vi "Controle_Manip_Main_GUI_Backup2.vi"() -> ()   [LabVIEW 2019] (continued)
                  n486 = Index Array(array=w526, index=0) -> (element=w525:refnum<vi>)
                  n487 = property class="Page"(reference=w525, "PageVis"=w524) -> ()  [unwired: 1 in, 2 out]
                }
              }
            }
            frame #13 {
              # "Advance progress bar"
              n488 = local write "Scan Main Progess Bar"(u8 70 ("Scan Main Progess Bar")) -> ()
            }
            frame #14 {
              # "PZA12 Fine Delay Translation Stage"
              n489 = case shown="True" "PZC200 On?" {
                frame False {
                  n490 = local read "Scan Contrast Ctrls"() -> (w571:refnum<vi>[])
                  n491 = local read "ESP 301 On?"() -> (w570:bool)
                  n492 = call "Enable&Disable_Controls.vi"("Enum"=enum16{"Enabled", "Disabled", "Disabled&Grayed"}."Disabled&Grayed", "References"=w571) -> ()  [unwired: 1 in]
                  n493 = case shown="True" w570 {
                    frame True {
                      n494 = property on="Experimental parameters tab" class="TabCtl (strict)" props=["Pages", "Value"]() -> ("Pages"=w576:refnum<vi>[])  [unwired: 2 in, 3 out]
                      n495 = property on="Experiment Graph Controls" class="TabCtl (strict)" props=["Value", "Pages"]() -> ("Pages"=w577:refnum<vi>[])  [unwired: 2 in, 3 out]
                      n496 = Index Array(array=w576, index=3) -> (element=w575:refnum<vi>)
                      n497 = Index Array(array=w577, index=3) -> (element=w579:refnum<vi>)
                      n498 = property class="Page"(reference=w575, "PageVis"=TRUE ("Page Visible")) -> ()  [unwired: 1 in, 2 out]
                      n499 = property class="Page"(reference=w579, "PageVis"=TRUE ("Page Visible")) -> ()  [unwired: 1 in, 2 out]
                    }
                    frame False {
                      n500 = property on="Experimental parameters tab" class="TabCtl (strict)"() -> ("Pages"=w584:refnum<vi>[])  [unwired: 2 in, 2 out]
                      n501 = property on="Experiment Graph Controls" class="TabCtl (strict)" props=["Value", "Pages"]() -> ("Pages"=w585:refnum<vi>[])  [unwired: 2 in, 3 out]
                      n502 = Index Array(array=w584, index=3) -> (element=w583:refnum<vi>)
                      n503 = Index Array(array=w585, index=3) -> (element=w587:refnum<vi>)
                      n504 = property class="Page"(reference=w583, "PageVis"=FALSE ("Page Visible")) -> ()  [unwired: 1 in, 2 out]
                      n505 = property class="Page"(reference=w587, "PageVis"=FALSE ("Page Visible")) -> ()  [unwired: 1 in, 2 out]
                    }
                  }
                }
                frame True {
                  n506 = stacked-sequence {
                    frame #0 {
                      w604 = TRUE
                      w603 = FALSE
                      n507 = property on="Experiment Graph Controls" class="TabCtl (strict)"("Value"=T25."Contrast" ("Experiment Graph Controls")) -> ("Pages"=w599:refnum<vi>[])  [unwired: 2 in, 2 out]
                      n508 = property on="Experimental parameters tab" class="TabCtl (strict)"("Value"=T19."Translation" ("Experimental parameters tab")) -> ("Pages"=w598:refnum<vi>[])  [unwired: 2 in, 2 out]
                      n509 = local read "Log file"() -> (w594:string)
                      n510 = Index Array(array=w599, index=3) -> (element=w601:refnum<vi>)
                      n511 = Index Array(array=w598, index=3) -> (element=w595:refnum<vi>)
                      n512 = property class="Page"(reference=w601, "PageVis"=TRUE ("Page Visible")) -> ()  [unwired: 1 in, 2 out]
                      n513 = property on="Stop Contrast" class="Bool (strict)"("Visible"=w603) -> ()  [unwired: 2 in, 2 out]
                      n514 = property on="Pause Contrast" class="Bool (strict)"("Visible"=w603) -> ()  [unwired: 2 in, 2 out]
                      n515 = property class="Page"(reference=w595, "PageVis"=TRUE ("Page Visible")) -> ()  [unwired: 1 in, 2 out]
                      n516 = call "Write2LogFile.vi"("Add to log file"="Initialise communication with PZC", "Log file before"=w594, "Checkbox"=FALSE) -> ("Log file after"=w593:string)
                      n517 = local write "Log file"(w593) -> ()
                      n518 = local read "Scan Contrast Ctrls"() -> (w606:refnum<vi>[])
                      n519 = property on="Save Contrast" class="Bool (strict)"("Visible"=w604) -> ()  [unwired: 2 in, 2 out]
                      n520 = property on="Acquire Contrast" class="Bool (strict)"("Visible"=w604) -> ()  [unwired: 2 in, 2 out]
                      n521 = call "Enable&Disable_Controls.vi"("Enum"=enum16{"Enabled", "Disabled", "Disabled&Grayed"}."Enabled", "References"=w606) -> ()  [unwired: 1 in]
                    }
                    frame #1 {
                      # "RS232/10"
                      n522 = local read "PZC200 COM Port"() -> (w608:dbl)
                      n523 = call "Create Instrument Channel.vi"("XON/XOFF Handshaking(F)"=TRUE, "Baud Rate (38400)"=u32 19200, "COM Port (1)"=w608, "(T) - GPIB, F - RS232"=FALSE) -> ("Instrument Channel out"=w612:string)  [unwired: 5 in, 2 out]
                      n524 = call "SendCommand.vi"("Command"="1TS?", "Instrument Channel"=w612) -> ("Instrument Channel out"=w613:string)  [unwired: 8 in, 1 out]
                      n525 = call "ReadCommand.vi"("Disable MAV check (F)"=TRUE, "Instrument Channel"=w613) -> ("Response"=w614:string, "Instrument Channel out"=w607:string)  [unwired: 7 in, 1 out]
                      "Response" <- w614
                      n526 = String Length(string=w614) -> (length=w621:i32)
                      n527 = Subtract(x=w621, y=1) -> (x-y=w619:i32)
                      n528 = local write "PZC200 Instrument Channel"(w607) -> ()
                      n529 = String Subset(string=w614, offset (0)=w619) -> (substring=w618:string)  [unwired: 1 in]
                      n530 = case shown="\"@\", Default" w618 {
                        tunnel: [FALSE TRUE TRUE] -> w617
                        frame "@", Default {
                        }
                        frame "Q" {
                        }
                        frame "P" {
                        }
                      }
                      n531 = local write "LinTFine Motor On?"(w617) -> ()
                      n532 = call "PZCGetPos.vi"("Instrument Channel"=w607) -> ("Position"=w615:i32)  [unwired: 1 in, 2 out]
                      n533 = local write "PZC Position Readout (usteps)"(w615) -> ()
                    }
                  }
                }
              }
            }
            frame #15 {
              # "Advance progress bar"
              n534 = local write "Scan Main Progess Bar"(u8 85 ("Scan Main Progess Bar")) -> ()
            }
            frame #16 {
              # "Attocube ANC350 with 2 ANPx51 and 1 ANPz51"
              n535 = case shown="True" "Attocubes On?" {
                tunnel: [FALSE ("Page Visible") TRUE] -> w627
                frame False {
                }
                frame True {
                  n536 = stacked-sequence {
                    frame #0 {
                      n537 = control-ref of="Experimental parameters tab"() -> (w637:refnum<vi>)
                      n538 = property class="TabCtl (strict)"(reference=w637, "Value"=T19."Microscope objective") -> ()  [unwired: 1 in, 2 out]
                      n539 = local read "Log file"() -> (w641:string)
                      n540 = control-ref of="Tab Objective Sample"() -> (w639:refnum<vi>)
                      n541 = call "Write2LogFile.vi"("Add to log file"="Initialise communication with ANC350", "Log file before"=w641, "Checkbox"=FALSE) -> ("Log file after"=w642:string)
                      n542 = local write "Log file"(w642) -> ()
                      n543 = property class="TabCtl (strict)"(reference=w639, "Value"=T22."Sample piezo stack") -> ()  [unwired: 1 in, 2 out]
                      "ourDLL" <- path "C:/Users/manip/Documents/Controle_Manip_2020/subVIs/Attocubes/anc350v4.dll"
                    }
                    frame #1 {
                      w647 = u32 1 items=["None", "USB", "TCP", "All"] ("Interface types")
                      n544 = local read "ourDLL"() -> (w644:path)
                      n545 = call "ANC350v4_Discover.vi"("Path to *.DLL"=w644, "Interface types"=w647) -> ("ANC350v4 found"=w646:u32, "error ANC350v4_discover"=w645:errorcluster)  [unwired: 12 in]
                      n546 = case shown="1" w646 {
                        tunnel: w645 -> [_ w649]
                        tunnel: w644 -> [_ w648]
                        frame 0, Default {
                        }
                        frame 1 {
                          n547 = stacked-sequence {
                            seq-local: [w651 _] -> [_ w682]
                            seq-local: [w650 _] -> [_ w681]
                            tunnel: w649 -> [w668 _]
                            tunnel: w648 -> [w657 w680]
                            frame #0 {
                              w652 = u8 0 items=["1", "2", "3"] ("axis")
                              w655 = u8 2 items=["1", "2", "3"] ("axis")
                              w656 = u8 1 items=["1", "2", "3"] ("axis")
                              n548 = call "ANC350v4sub_Connect.vi"("Path to *.DLL"=w657, "deviceNumber"=0, "error in"=w668) -> ("ANC350v4_Handle_Out"=w664:u64, "error ANC350v4_Dis/Connect"=w667:errorcluster)  [unwired: 11 in]
                              n549 = call "ANC350v4_GetDeviceInfo.vi"("Path to *.DLL"=w657, "deviceNumber"=u32 0, "error in"=w667) -> ("connected"=→"ANC connected":bool, "Error_ANC350v4_getDeviceInfo"=w663:errorcluster)  [unwired: 5 in, 6 out]
                              n550 = call "ANC350v4_GetPosition.vi"("deviceHandle"=w664, "Path to *.DLL"=w657, "axis"=w652, "error in"=w663) -> ("deviceHandle"=w661:u64, "Position [µm | m°]"=w662:dbl, "error ANC350v4_getPosition"=w660:errorcluster)  [unwired: 8 in, 1 out]
                              n551 = local write "Att Pos Y"(w662) -> ()
                              n552 = call "ANC350v4_GetPosition.vi"("deviceHandle"=w661, "Path to *.DLL"=w657, "axis"=w656, "error in"=w660) -> ("deviceHandle"=w659:u64, "Position [µm | m°]"=w653:dbl, "error ANC350v4_getPosition"=w658:errorcluster)  [unwired: 8 in, 1 out]
                              n553 = local write "Att Pos X"(w653) -> ()
                              n554 = call "ANC350v4_GetPosition.vi"("deviceHandle"=w659, "Path to *.DLL"=w657, "axis"=w655, "error in"=w658) -> ("deviceHandle"=w651:u64, "Position [µm | m°]"=w654:dbl, "error ANC350v4_getPosition"=w650:errorcluster)  [unwired: 8 in, 1 out]
                              n555 = local write "Att Pos Z"(w654) -> ()
                            }
                            frame #1 {
                              w670 = u8 2 items=["1", "2", "3"] ("axis")
                              w671 = u8 1 items=["1", "2", "3"] ("axis")
                              w672 = u8 0 items=["1", "2", "3"] ("axis")
                              w679 = 0.1 ("TargetRange [µm | m°]")
                              # "Define Target resolution in um"
                              n556 = call "ANC350v4_SetTargetRange.vi"("deviceHandle"=w682, "Path to *.DLL"=w680, "axis"=w672, "TargetRange [µm | m°]"=w679, "error in"=w681) -> ("deviceHandle"=w678:u64, "error ANC350v4_setTargetRange"=w676:errorcluster)  [unwired: 8 in, 1 out]
                              n557 = call "ANC350v4_SetTargetRange.vi"("deviceHandle"=w678, "Path to *.DLL"=w680, "axis"=w671, "TargetRange [µm | m°]"=w679, "error in"=w676) -> ("deviceHandle"=w677:u64, "error ANC350v4_setTargetRange"=w675:errorcluster)  [unwired: 8 in, 1 out]
                              n558 = call "ANC350v4_SetTargetRange.vi"("deviceHandle"=w677, "Path to *.DLL"=w680, "axis"=w670, "TargetRange [µm | m°]"=w679, "error in"=w675) -> ("deviceHandle"=→"Att DeviceHandle":u64, "error ANC350v4_setTargetRange"=→"Att Error":errorcluster)  [unwired: 8 in, 1 out]
                            }
                          }
                        }
                      }
                    }
                  }
                }
              }
              n559 = control-ref of="Tab Objective Sample"() -> (w629:refnum<vi>)
              n560 = property class="TabCtl (strict)"(reference=w629) -> ("Pages"=w630:refnum<vi>[])  [unwired: 1 in, 2 out]
              n561 = Index Array(array=w630, index=1) -> (element=w631:refnum<vi>)
              n562 = property class="Page"(reference=w631, "PageVis"=w627) -> ()  [unwired: 1 in, 2 out]
            }
            frame #17 {
              # "Montana Cryostation s50"
              n563 = case shown="True" "Cryostation On?" {
                frame False {
                }
                frame True {
                  w698 = 10.0 ("y")
                  n564 = call "CryoConnect.vi"() -> ("connection ID"=w688:refnum<k5>)
                  "Cryostation ID" <- w688
                  n565 = local read "Log file"() -> (w687:string)
                  n566 = call "Write2LogFile.vi"("Add to log file"="Initialise communication with Cryostation", "Log file before"=w687, "Checkbox"=FALSE) -> ("Log file after"=w686:string)
                  n567 = local write "Log file"(w686) -> ()
                  n568 = call "GetCryoInfo.vi"("connection ID"=w688) -> ("User Stability"=w693:dbl, "User Temp"=w692:dbl, "connection ID out"=w694:refnum<k5>, "Sample Stability"=w691:dbl, "Sample Temp"=w695:dbl, "Platform Stability"=w690:dbl, "Platform Temp"=w689:dbl)  [unwired: 4 in]
                  n569 = local write "Cryo Platform Temp"(w689) -> ()
                  n570 = Multiply(x=w695, y=w698) -> (x*y=w696:dbl)
                  n571 = local write "Cryo Sample Stability"(w691) -> ()
                  n572 = local write "Cryostation ID"(w694) -> ()
                  n573 = local write "Cryo User Stability"(w693) -> ()
                  n574 = local write "Cryo Sample Temp"(w695) -> ()
                  n575 = local write "Cryo Platform Stability"(w690) -> ()
                  n576 = local write "Cryo User Temp"(w692) -> ()
                  n577 = Round To Nearest(number=w696) -> (nearest integer value=w697:dbl)
                  n578 = Divide(x=w697, y=w698) -> (x/y=w699:dbl)
                  n579 = local write "Temperature (K)"(w699) -> ()
                }
              }
            }
            frame #18 {
              # "PicoHarp"
              n580 = case shown="True" "PicoHarp On?" {
                frame False {
                  n581 = local write "Connected"(FALSE) -> ()
                }
                frame True {
                  n582 = local read "Log file"() -> (w711:string)
                  n583 = property on="Experiment Graph Controls" class="TabCtl (strict)"("Value"=T25."APDs" ("Experiment Graph Controls")) -> ("Pages"=w706:refnum<vi>[])  [unwired: 2 in, 2 out]
                  n584 = call "Write2LogFile.vi"("Add to log file"="Initialise communication with PicoHarp", "Log file before"=w711, "Checkbox"=FALSE) -> ("Log file after"=w710:string)
                  n585 = call "PH_Init.vi"() -> ("PH_Init_Data"=→"PH_Init_Data":T11)
                  n586 = local write "Log file"(w710) -> ()
                  n587 = Index Array(array=w706, index=4) -> (element=w707:refnum<vi>)
                  n588 = property class="Page"(reference=w707, "PageVis"=TRUE ("Page Visible")) -> ()  [unwired: 1 in, 2 out]
                  n589 = local write "Connected"(TRUE) -> ()
                }
              }
            }
            frame #19 {
              # "Final activation message"
              n590 = local read "Log file"() -> (w717:string)
              n591 = property on="Experiment Graph Controls" class="TabCtl (strict)"("Value"=T25."Settings" ("Experiment Graph Controls")) -> ()  [unwired: 2 in, 2 out]
              n592 = call "Write2LogFile.vi"("Add to log file"="All devices activated !", "Log file before"=w717, "Checkbox"=FALSE) -> ("Log file after"=w718:string)
              n593 = local write "Log file"(w718) -> ()
              n594 = local write "Scan Main Progess Bar"(u8 100 ("Scan Main Progess Bar")) -> ()
            }
            frame #20 {
              # "Autosave Init"
              n595 = local read "Auto< ?"() -> (w719:bool)
              n596 = case shown="True" w719 {
                frame False {
                  w720 = TRUE ("Visible")
                  n597 = property on="Save Spectrum N" class="Bool (strict)"("Visible"=w720) -> ()  [unwired: 2 in, 2 out]
                  n598 = property on="Save XY Map" class="Bool (strict)"("Visible"=w720) -> ()  [unwired: 2 in, 2 out]
                  n599 = property on="Save Spectrum" class="Bool (strict)"("Visible"=w720) -> ()  [unwired: 2 in, 2 out]
                  n600 = property on="Save PLE" class="Bool (strict)"("Visible"=w720) -> ()  [unwired: 2 in, 2 out]
                  n601 = property on="Save fPow" class="Bool (strict)"("Visible"=w720) -> ()  [unwired: 2 in, 2 out]
                  n602 = property on="Save Custom Diode Spectrum" class="Bool (strict)"("Visible"=w720) -> ()  [unwired: 2 in, 2 out]
                  n603 = property on="Save Michelson" class="Bool (strict)"("Visible"=w720) -> ()  [unwired: 2 in, 2 out]
                  n604 = property on="Save Polarisation" class="Bool (strict)"("Visible"=w720) -> ()  [unwired: 2 in, 2 out]
                  n605 = property on="Save Contrast" class="Bool (strict)"("Visible"=w720) -> ()  [unwired: 2 in, 2 out]
                }
                frame True {
                  w721 = FALSE ("Visible")
                  n606 = property on="Save Spectrum N" class="Bool (strict)"("Visible"=w721) -> ()  [unwired: 2 in, 2 out]
                  n607 = property on="Save XY Map" class="Bool (strict)"("Visible"=w721) -> ()  [unwired: 2 in, 2 out]
                  n608 = property on="Save Spectrum" class="Bool (strict)"("Visible"=w721) -> ()  [unwired: 2 in, 2 out]
                  n609 = property on="Save PLE" class="Bool (strict)"("Visible"=w721) -> ()  [unwired: 2 in, 2 out]
                  n610 = property on="Save fPow" class="Bool (strict)"("Visible"=w721) -> ()  [unwired: 2 in, 2 out]
                  n611 = property on="Save Polarisation" class="Bool (strict)"("Visible"=w721) -> ()  [unwired: 2 in, 2 out]
                  n612 = property on="Save Michelson" class="Bool (strict)"("Visible"=w721) -> ()  [unwired: 2 in, 2 out]
                  n613 = property on="Save Contrast" class="Bool (strict)"("Visible"=w721) -> ()  [unwired: 2 in, 2 out]
                  n614 = property on="Save Custom Diode Spectrum" class="Bool (strict)"("Visible"=w721) -> ()  [unwired: 2 in, 2 out]
                }
              }
            }
          }
        }
      }
    }
    frame #2 {
      # "Main Program"
      n615 = while {
        stop <- w873 stop-if-true
        # "Main loop with unique event structure handling nearly all events"
        n616 = event shown="[50] \"Fit?\": Mouse Down" {
          selector: _ -> [_ _ _ _ _ _ _ _ _ _ _ _ _ _ _ _ _ _ _ _ _ _ _ _ _ _ _ _ _ _ _ _ _ _ _ _ _ _ _ _ _ _ _ _ _ _ _ _ _ _ _ _ _ _]
          dyn-events: _ -> [_ _ _ _ _ _ _ _ _ _ _ _ _ _ _ _ _ _ _ _ _ _ _ _ _ _ _ _ _ _ _ _ _ _ _ _ _ _ _ _ _ _ _ _ _ _ _ _ _ _ _ _ _ _]
          timeout: 500 -> [_ _ _ _ _ _ _ _ _ _ _ _ _ _ _ _ _ _ _ _ _ _ _ _ _ _ _ _ _ _ _ _ _ _ _ _ _ _ _ _ _ _ _ _ _ _ _ _ _ _ _ _ _ _]
          tunnel: [_ _ _ _ _ _ _ _ _ _ _ _ _ _ _ _ _ _ _ _ _ _ _ _ _ _ _ _ _ _ _ _ _ _ _ _ _ _ _ _ _ _ _ _ _ _ _ _ w4486 _ _ _ _ _] -> w873
          event "Acquire Time Trace", "Acquire Polarisation", "Acquire XY Map", "Acquire Contrast", "Acquire Michelson", "Acquire Spectrum", "Fast Acq", "Acquire Custom Diode Spectrum", "Acquire fPow", "Acquire PLE": Mouse Down {
            # "FAILLE\naucune protection \nde teigger si ESP et \nPicoHarp mais pas LF"
            # "Launch an acquisition or an experiment"
            n617 = event-data() -> ("CtlRef"=w879:refnum<vi>)  [unwired: 1 in, 7 out]
            n618 = local read "LightField On?"() -> (w876:bool)
            n619 = local read "PicoHarp On?"() -> (w877:bool)
            n620 = local read "ESP 300 On?"() -> (w878:bool)
            n621 = And(x=w878, y=w877) -> (x .and. y?=w875:bool)
            n622 = Or(x=w876, y=w875) -> (x .or. y?=w874:bool)
            n623 = stacked-sequence {
              tunnel: w879 -> [w881 w2777]
              tunnel: w874 -> [w880 _]
              frame #0 {
                # "Actual measurements"
                n624 = case shown="True" w880 {
                  tunnel: w881 -> [_ w886]
                  frame False {
                    n625 = local read "Log file"() -> (w885:string)
                    n626 = call "Write2LogFile.vi"("Add to log file"="LightField not activated; cannot acquire", "Log file before"=w885, "Checkbox"=FALSE) -> ("Log file after"=w884:string)
                    n627 = local write "Log file"(w884) -> ()
                  }
                  frame True {
                    n628 = property class="Bool"(reference=w886) -> ("Label.Text"=w887:string)  [unwired: 1 in, 2 out]
                    n629 = case shown="\"Acquire PLE\"" w887 {
                      frame "Acquire Spectrum", Default {
                        n630 = stacked-sequence {
                          frame #0 {
                            # "background"
                            n631 = local read "Background taken?"() -> (w888:bool)
                            n632 = case shown="False" w888 {
                              frame False {
                                n633 = stacked-sequence {
                                tunnel: [_ _ w934] -> w889
                                frame #0 {
                                n634 = property on="CCD 1D Spectrum Main" class="XYGraph (strict)"("YScale.Offset"=0.0 ("Y Scale.Offset and Multiplier:Offset")) -> ()  [unwired: 2 in, 2 out]
                                }
                                frame #1 {
                                # "make sure shutter is closed"
                                n635 = local read "KCube Shutter On?"() -> (w920:bool)
                                n636 = control-ref of="Shutter Ctrls"() -> (w924:refnum<vi>)
                                n637 = property class="Ring (strict)"(reference=w924) -> ("Value"=w923:u16)  [unwired: 1 in, 2 out]
                                n638 = control-ref of="KCube Shutter Device Reference"() -> (w925:refnum<vi>)
                                n639 = Equal?(x=w923, y=u16 0) -> (x = y?=w921:bool)
                                n640 = case shown="False" w921 {
                                tunnel: w925 -> [w928 _]
                                tunnel: w924 -> [w927 _]
                                tunnel: w920 -> [w926 _]
                                frame False {
                                n641 = call "Shutter.vi"("KCube Shutter Device Reference 2"=w928, "Shutter Ctrls 2"=w927, "Shutter on?"=w926) -> ()
                                }
                                frame True {
                                }
                                }
                                }
                                frame #2 {
                                # "acquire"
                                n642 = local read "LightField Automation error out"() -> (w932:errorcluster)
                                n643 = local read "LightField Automation out"() -> (w933:refnum<class "LightField Automation.lvclass">)
                                n644 = local read "Accumulations"() -> (w929:dbl)
                                n645 = call "LFA_Capture.vi"("error in (no error)"=w932, "Frames"=w929, "LightField Automation in"=w933) -> ("error out"=w931:errorcluster, "Data"=w934:T26, "LightField Automation out"=w930:refnum<class "LightField Automation.lvclass">)  [unwired: 6 in]
                                n646 = local write "LightField Automation error out"(w931) -> ()
                                n647 = local write "LightField Automation out"(w930) -> ()
                                }
                                }
                                n648 = local read "Acq Mode"() -> (w890:T3)
                                n649 = case shown="\"Spectrum\", Default" w890 {
                                selector: w890 -> [w891 w909]
                                tunnel: w889 -> [w892 w910]
                                frame "Spectrum", Default {
                                n650 = stacked-sequence {
                                tunnel: w892 -> [_ w903 _ _]
                                tunnel: w891 -> [_ w901 _ _]
                                frame #0 {
                                n651 = property on="CCD 2D Image Main" class="IntGraph (strict)"("Visible"=FALSE) -> ()  [unwired: 2 in, 2 out]
                                n652 = property on="CCD 1D Spectrum Main" class="XYGraph (strict)"("Visible"=TRUE) -> ()  [unwired: 2 in, 2 out]
                                }
                                frame #1 {
                                n653 = local read "Wavelength calibration"() -> (w900:dbl[])
                                n654 = local read "CCD ROI"() -> (w896:T20)
                                n655 = Divide(x=1239.842, y=w900) -> (x/y=w898:dbl[])
                                n656 = call "PrepareData4Graph.vi"("Wavelength nm"=w898, "DataLF"=w903, "CCD ROI"=w896, "AcqMode"=w901, "Data type"=T30."Spectre") -> ("Spectrum"=w902:cluster{"Array 2":dbl[], "Array":dbl[]}, "PLInt out"=w895:dbl[])  [unwired: 2 in, 2 out]
                                n657 = local write "CCD 1D Spectrum Main"(w902) -> ()
                                n658 = local write "BackgroundSpec"(w895) -> ()
                                }
                                frame #2 {
                                n659 = local read "BackgroundSpec"() -> (w904:dbl[])
                                n660 = call-poly <vilib>:"Mean.vi"("X"=w904) -> ("mean"=w906:dbl)  [unwired: 1 out]
                                n661 = Negate(x=w906) -> (-x=w905:dbl)
                                n662 = property on="CCD 1D Spectrum Main" class="XYGraph (strict)"("YScale.Offset"=w905) -> ()  [unwired: 2 in, 2 out]
                                }
                                frame #3 {
                                n663 = local write "Background taken?"(TRUE ("Background taken?")) -> ()
                                n664 = property on="Background substract" class="Enum (strict)"("Value"=enum16{"None", "Shutter"}."None" ("Background substract")) -> ()  [unwired: 2 in, 2 out]
                                }
                                }
                                }
                                frame "Image" {
                                n665 = stacked-sequence {
                                tunnel: w910 -> [_ w918]
                                tunnel: w909 -> [_ w916]
                                frame #0 {
                                n666 = property on="CCD 1D Spectrum Main" class="XYGraph (strict)"("Visible"=FALSE) -> ()  [unwired: 2 in, 2 out]
                                n667 = property on="CCD 2D Image Main" class="IntGraph (strict)"("Visible"=TRUE) -> ()  [unwired: 2 in, 2 out]
                                }
                                frame #1 {
                                n668 = local read "Wavelength calibration"() -> (w917:dbl[])
                                n669 = local read "CCD ROI"() -> (w913:T20)
                                n670 = call "PrepareData4Graph.vi"("Wavelength nm"=w917, "DataLF"=w918, "CCD ROI"=w913, "AcqMode"=w916, "Data type"=T30."Spectre") -> ("Intensity Graph"=w915:dbl[][])  [unwired: 2 in, 3 out]
                                n671 = local write "CCD 2D Image Main"(w915) -> ()
                                }
                                }
                                }
                                }
                              }
                              frame True {
                              }
                            }
                          }
                          frame #1 {
                            # "measurement"
                            n672 = stacked-sequence {
                              frame #0 {
                                # "open shutter if closed"
                                n673 = control-ref of="KCube Shutter Device Reference"() -> (w937:refnum<vi>)
                                n674 = control-ref of="Shutter Ctrls"() -> (w936:refnum<vi>)
                                n675 = property class="Ring (strict)"(reference=w936) -> ("Value"=w938:u16)  [unwired: 1 in, 2 out]
                                n676 = local read "KCube Shutter On?"() -> (w941:bool)
                                n677 = Equal?(x=w938, y=u16 0) -> (x = y?=w940:bool)
                                n678 = property on="Experiment Graph Controls" class="TabCtl (strict)"("Value"=T25."Spectrum" ("Experiment Graph Controls")) -> ()  [unwired: 2 in, 2 out]
                                n679 = case shown="True" w940 {
                                tunnel: w937 -> [_ w944]
                                tunnel: w936 -> [_ w943]
                                tunnel: w941 -> [_ w942]
                                frame False {
                                }
                                frame True {
                                n680 = call "Shutter.vi"("KCube Shutter Device Reference 2"=w944, "Shutter Ctrls 2"=w943, "Shutter on?"=w942) -> ()
                                }
                                }
                              }
                              frame #1 {
                                # "set CCD ROI and acquire"
                                n681 = local read "LightField Automation error out"() -> (w953:errorcluster)
                                n682 = local read "LightField Automation out"() -> (w945:refnum<class "LightField Automation.lvclass">)
                                n683 = local read "CCD ROI"() -> (w952:T20)
                                n684 = local read "Accumulations"() -> (w949:dbl)
                                n685 = call "Adv_SetROI.vi"("error in (no error)"=w953, "ROI"=w952, "LightField Automation in"=w945) -> ("error out"=w950:errorcluster, "LightField Automation out"=w951:refnum<class "LightField Automation.lvclass">)  [unwired: 7 in]
                                n686 = call "LFA_Capture.vi"("error in (no error)"=w950, "Frames"=w949, "LightField Automation in"=w951) -> ("error out"=w948:errorcluster, "Data"=w947:T26, "LightField Automation out"=w946:refnum<class "LightField Automation.lvclass">)  [unwired: 6 in]
                                n687 = local write "LightField Automation out"(w946) -> ()
                                n688 = local write "LightField Automation error out"(w948) -> ()
                                n689 = local write "Data"(w947) -> ()
                              }
                              frame #2 {
                                # "close shutter"
                                n690 = local read "KCube Shutter On?"() -> (w956:bool)
                                n691 = control-ref of="KCube Shutter Device Reference"() -> (w955:refnum<vi>)
                                n692 = control-ref of="Shutter Ctrls"() -> (w954:refnum<vi>)
                                n693 = call "Shutter.vi"("KCube Shutter Device Reference 2"=w955, "Shutter Ctrls 2"=w954, "Shutter on?"=w956) -> ()
                              }
                              frame #3 {
                                # "Show data accordingly"
                                n694 = local read "Data"() -> (w957:T26)
                                n695 = local read "Acq Mode"() -> (w958:T3)
                                n696 = case shown="\"Spectrum\", Default" w958 {
                                selector: w958 -> [w959 w978]
                                tunnel: w957 -> [w960 w979]
                                frame "Spectrum", Default {
                                n697 = stacked-sequence {
                                tunnel: w960 -> [_ w976 _]
                                tunnel: w959 -> [_ w975 _]
                                frame #0 {
                                n698 = property on="CCD 1D Spectrum Main" class="XYGraph (strict)"("Visible"=TRUE) -> ()  [unwired: 2 in, 2 out]
                                n699 = property on="CCD 2D Image Main" class="IntGraph (strict)"("Visible"=FALSE) -> ()  [unwired: 2 in, 2 out]
                                }
                                frame #1 {
                                n700 = local read "Wavelength calibration"() -> (w974:dbl[])
                                n701 = local read "CCD ROI"() -> (w970:T20)
                                n702 = local read "BackgroundSpec"() -> (w964:dbl[])
                                n703 = Divide(x=1239.842, y=w974) -> (x/y=w972:dbl[])
                                n704 = call "PrepareData4Graph.vi"("BackgroundSpec"=w964, "Wavelength nm"=w972, "DataLF"=w976, "CCD ROI"=w970, "AcqMode"=w975, "Data type"=T30."Spectre") -> ("Spectrum"=w963:cluster{"Array 2":dbl[], "Array":dbl[]}, "PLInt out"=w968:dbl[])  [unwired: 1 in, 2 out]
                                n705 = control-ref of="Cnts"() -> (w969:refnum<vi>)
                                n706 = local read "Excitation Power (uW)"() -> (w966:dbl)
                                n707 = local write "CCD 1D Spectrum Main"(w963) -> ()
                                n708 = local read "Acq Time (ms)"() -> (w967:dbl)
                                n709 = local read "Display Mode"() -> (w965:u16)
                                n710 = call "2Cnts.vi"("Array Background"=w964, "Pow W"=w966, "AcqTime ms"=w967, "Cnts Ref"=w969, "Display Mode"=w965, "Array"=w968) -> ()  [unwired: 1 out]
                                }
                                frame #2 {
                                n711 = property on="Full scale" class="Bool (strict)"("Val(Sgnl)"=TRUE ("Value (Signaling)")) -> ()  [unwired: 2 in, 2 out]
                                }
                                }
                                }
                                frame "Image" {
                                n712 = stacked-sequence {
                                tunnel: w979 -> [_ w987]
                                tunnel: w978 -> [_ w985]
                                frame #0 {
                                n713 = property on="CCD 1D Spectrum Main" class="XYGraph (strict)"("Visible"=FALSE) -> ()  [unwired: 2 in, 2 out]
                                n714 = property on="CCD 2D Image Main" class="IntGraph (strict)"("Visible"=TRUE) -> ()  [unwired: 2 in, 2 out]
                                }
                                frame #1 {
                                n715 = local read "Wavelength calibration"() -> (w986:dbl[])
                                n716 = local read "CCD ROI"() -> (w982:T20)
                                n717 = call "PrepareData4Graph.vi"("Wavelength nm"=w986, "DataLF"=w987, "CCD ROI"=w982, "AcqMode"=w985, "Data type"=T30."Spectre") -> ("Intensity Graph"=w984:dbl[][])  [unwired: 2 in, 3 out]
                                n718 = local write "CCD 2D Image Main"(w984) -> ()
                                }
                                }
                                }
                                }
                              }
                            }
                          }
                        }
                      }
                      frame "Acquire fPow" {
                        n719 = stacked-sequence {
                          frame #0 {
                            # "background"
                            n720 = local read "Background taken?"() -> (w988:bool)
                            n721 = case shown="False" w988 {
                              frame False {
                                n722 = stacked-sequence {
                                tunnel: [_ _ w1034] -> w989
                                frame #0 {
                                n723 = property on="CCD 1D Spectrum Main" class="XYGraph (strict)"("YScale.Offset"=0.0 ("Y Scale.Offset and Multiplier:Offset")) -> ()  [unwired: 2 in, 2 out]
                                }
                                frame #1 {
                                # "make sure shutter is closed"
                                n724 = local read "KCube Shutter On?"() -> (w1020:bool)
                                n725 = control-ref of="Shutter Ctrls"() -> (w1024:refnum<vi>)
                                n726 = property class="Ring (strict)"(reference=w1024) -> ("Value"=w1023:u16)  [unwired: 1 in, 2 out]
                                n727 = control-ref of="KCube Shutter Device Reference"() -> (w1025:refnum<vi>)
                                n728 = Equal?(x=w1023, y=u16 0) -> (x = y?=w1021:bool)
                                n729 = case shown="False" w1021 {
                                tunnel: w1025 -> [w1028 _]
                                tunnel: w1024 -> [w1027 _]
                                tunnel: w1020 -> [w1026 _]
                                frame False {
                                n730 = call "Shutter.vi"("KCube Shutter Device Reference 2"=w1028, "Shutter Ctrls 2"=w1027, "Shutter on?"=w1026) -> ()
                                }
                                frame True {
                                }
                                }
                                }
                                frame #2 {
                                # "acquire"
                                n731 = local read "LightField Automation error out"() -> (w1032:errorcluster)
                                n732 = local read "LightField Automation out"() -> (w1033:refnum<class "LightField Automation.lvclass">)
                                n733 = local read "Accumulations"() -> (w1029:dbl)
                                n734 = call "LFA_Capture.vi"("error in (no error)"=w1032, "Frames"=w1029, "LightField Automation in"=w1033) -> ("error out"=w1031:errorcluster, "Data"=w1034:T26, "LightField Automation out"=w1030:refnum<class "LightField Automation.lvclass">)  [unwired: 6 in]
                                n735 = local write "LightField Automation error out"(w1031) -> ()
                                n736 = local write "LightField Automation out"(w1030) -> ()
                                }
                                }
                                n737 = local read "Acq Mode"() -> (w990:T3)
                                n738 = case shown="\"Spectrum\", Default" w990 {
                                selector: w990 -> [w991 w1009]
                                tunnel: w989 -> [w992 w1010]
                                frame "Spectrum", Default {
                                n739 = stacked-sequence {
                                tunnel: w992 -> [_ w1003 _ _]
                                tunnel: w991 -> [_ w1001 _ _]
                                frame #0 {
                                n740 = property on="CCD 2D Image Main" class="IntGraph (strict)"("Visible"=FALSE) -> ()  [unwired: 2 in, 2 out]
                                n741 = property on="CCD 1D Spectrum Main" class="XYGraph (strict)"("Visible"=TRUE) -> ()  [unwired: 2 in, 2 out]
                                }
                                frame #1 {
                                n742 = local read "Wavelength calibration"() -> (w1000:dbl[])
                                n743 = local read "CCD ROI"() -> (w996:T20)
                                n744 = Divide(x=1239.842, y=w1000) -> (x/y=w998:dbl[])
                                n745 = call "PrepareData4Graph.vi"("Wavelength nm"=w998, "DataLF"=w1003, "CCD ROI"=w996, "AcqMode"=w1001, "Data type"=T30."Spectre") -> ("Spectrum"=w1002:cluster{"Array 2":dbl[], "Array":dbl[]}, "PLInt out"=w995:dbl[])  [unwired: 2 in, 2 out]
                                n746 = local write "CCD 1D Spectrum Main"(w1002) -> ()
                                n747 = local write "BackgroundSpec"(w995) -> ()
                                }
                                frame #2 {
                                n748 = local read "BackgroundSpec"() -> (w1004:dbl[])
                                n749 = call-poly <vilib>:"Mean.vi"("X"=w1004) -> ("mean"=w1006:dbl)  [unwired: 1 out]
                                n750 = Negate(x=w1006) -> (-x=w1005:dbl)
                                n751 = property on="CCD 1D Spectrum Main" class="XYGraph (strict)"("YScale.Offset"=w1005) -> ()  [unwired: 2 in, 2 out]
                                }
                                frame #3 {
                                n752 = local write "Background taken?"(TRUE ("Background taken?")) -> ()
                                n753 = property on="Background substract" class="Enum (strict)"("Value"=enum16{"None", "Shutter"}."None" ("Background substract")) -> ()  [unwired: 2 in, 2 out]
                                }
                                }
                                }
                                frame "Image" {
                                n754 = stacked-sequence {
                                tunnel: w1010 -> [_ w1018]
                                tunnel: w1009 -> [_ w1016]
                                frame #0 {
                                n755 = property on="CCD 1D Spectrum Main" class="XYGraph (strict)"("Visible"=FALSE) -> ()  [unwired: 2 in, 2 out]
                                n756 = property on="CCD 2D Image Main" class="IntGraph (strict)"("Visible"=TRUE) -> ()  [unwired: 2 in, 2 out]
                                }
                                frame #1 {
                                n757 = local read "Wavelength calibration"() -> (w1017:dbl[])
                                n758 = local read "CCD ROI"() -> (w1013:T20)
                                n759 = call "PrepareData4Graph.vi"("Wavelength nm"=w1017, "DataLF"=w1018, "CCD ROI"=w1013, "AcqMode"=w1016, "Data type"=T30."Spectre") -> ("Intensity Graph"=w1015:dbl[][])  [unwired: 2 in, 3 out]
                                n760 = local write "CCD 2D Image Main"(w1015) -> ()
                                }
                                }
                                }
                                }
                              }
                              frame True {
                              }
                            }
                          }
                          frame #1 {
                            w1040 = TRUE ("Visible")
                            w1041 = FALSE ("Visible")
                            # "init"
                            n761 = control-ref of="N Step Power  Diode Current (A)"() -> (w1044:refnum<vi>)
                            n762 = control-ref of="End Power  Diod Current (A)"() -> (w1045:refnum<vi>)
                            n763 = control-ref of="Start Power Diod Current (A)"() -> (w1046:refnum<vi>)
                            n764 = control-ref of="Acquire fPow"() -> (w1050:refnum<vi>)
                            n765 = control-ref of="Save fPow"() -> (w1048:refnum<vi>)
                            n766 = Build Array(w1050, w1048, w1046, w1045, w1044) -> (w1049:refnum<vi>[])
                            n767 = property on="Elapsed (s)" class="DigNum (strict)"("Visible"=TRUE) -> ()  [unwired: 2 in, 2 out]
                            n768 = call "Enable&Disable_Controls.vi"("Enum"=enum16{"Enabled", "Disabled", "Disabled&Grayed"}."Disabled&Grayed", "References"=w1049) -> ()  [unwired: 1 in]
                            n769 = control-ref of="MasterStop"() -> (w1038:refnum<vi>)
                            n770 = control-ref of="MasterPause"() -> (w1039:refnum<vi>)
                            n771 = control-ref of="Acquire fPow"() -> (w1043:refnum<vi>)
                            n772 = control-ref of="Save fPow"() -> (w1042:refnum<vi>)
                            n773 = property class="Bool (strict)"(reference=w1043, "Visible"=w1041) -> ()  [unwired: 1 in, 2 out]
                            n774 = property class="Bool (strict)"(reference=w1042, "Visible"=w1041) -> ()  [unwired: 1 in, 2 out]
                            n775 = property class="Bool (strict)"(reference=w1038, "Visible"=w1040) -> ()  [unwired: 1 in, 2 out]
                            n776 = property class="Bool (strict)"(reference=w1039, "Visible"=w1040) -> ()  [unwired: 1 in, 2 out]
                            n777 = property on="CCD 2D Image Main" class="IntGraph (strict)"("Visible"=FALSE) -> ()  [unwired: 2 in, 2 out]
                            n778 = property on="CCD 1D Spectrum Main" class="XYGraph (strict)"("Visible"=TRUE) -> ()  [unwired: 2 in, 2 out]
                          }
                          frame #2 {
                            # "measurement"
                            n779 = local read "N Step Power  Diode Current (A)"() -> (w1057:i32)
                            n780 = local read "End Power  Diod Current (A)"() -> (w1061:dbl)
                            n781 = Increment(x=w1057) -> (x+1=w1058:i32)
                            n782 = local read "Start Power Diod Current (A)"() -> (w1059:dbl)
                            n783 = Subtract(x=w1061, y=w1059) -> (x-y=w1060:dbl)
                            n784 = Divide(x=w1060, y=w1057) -> (x/y=w1056:dbl)
                            n785 = for {
                              N: w1058 -> [w1068]
                              tunnel: w1059 -> [w1075]
                              tunnel: w1056 -> [w1074]
                              shift-right: [w1072] -> w1052
                              shift-left: i32[][] [] -> [w1071]
                              shift-right: [w1069] -> w1054
                              shift-left: dbl[] [] -> [w1070]
                              i -> [w1064]
                              stop <- w1062 stop-if-true
                              n786 = Multiply(x=w1064, y=w1074) -> (x*y=w1076:dbl)
                              n787 = Add(x=w1075, y=w1076) -> (x+y=w1073:dbl)
                              n788 = Increment(x=w1064) -> (x+1=w1063:i32)
                              n789 = Divide(x=w1063, y=w1068) -> (x/y=w1067:dbl)
                              n790 = Multiply(x=w1067, y=100.0) -> (x*y=w1065:dbl)
                              n791 = stacked-sequence {
                                tunnel: w1073 -> [w1080 _ _ _ _ _]
                                tunnel: w1071 -> [_ _ _ _ w1137 _]
                                tunnel: [_ _ _ _ w1135 _] -> w1072
                                tunnel: w1070 -> [w1079 _ _ _ _ _]
                                tunnel: [w1077 _ _ _ _ _] -> w1069
                                tunnel: w1065 -> [_ _ _ _ _ w1179]
                                frame #0 {
                                # "set power and wait a bit"
                                n792 = local read "Photodiode handle out"() -> (w1083:refnum<visa-resource-name>)
                                n793 = local read "Photodiode error out"() -> (w1084:errorcluster)
                                n794 = local read "Diode Driver Error"() -> (w1082:errorcluster)
                                n795 = local read "DDE"() -> (w1081:refnum<visa-resource-name>)
                                n796 = stacked-sequence {
                                seq-local: [w1093 _ _] -> [_ _ w1112]
                                seq-local: [w1092 _ _] -> [_ _ w1111]
                                tunnel: w1081 -> [w1097 _ _]
                                tunnel: w1082 -> [w1090 _ _]
                                tunnel: [_ _ w1112] -> w1086
                                tunnel: [_ _ w1111] -> w1088
                                tunnel: w1083 -> [_ _ w1110]
                                tunnel: w1084 -> [_ _ w1109]
                                tunnel: [_ _ w1108] -> w1087
                                tunnel: [_ _ w1107] -> w1085
                                tunnel: w1080 -> [w1089 _ _]
                                tunnel: [_ _ w1106] -> w1078
                                frame #0 {
                                n797 = call <instrlib>:"TL4000 Get Laser Diode Current Setpoint.vi"("error in (no error)"=w1090, "instrument handle"=w1097) -> ("error out"=w1094:errorcluster, "Laser Diode Current Setpoint"=w1096:dbl, "instrument handle out"=w1095:refnum<visa-resource-name>)  [unwired: 7 in]
                                n798 = Not Equal?(x=w1089, y=w1096) -> (x != y?=w1091:bool)
                                n799 = case shown="True" w1091 {
                                tunnel: w1095 -> [w1099 w1104]
                                tunnel: w1094 -> [w1098 w1103]
                                tunnel: [w1099 w1102] -> w1093
                                tunnel: [w1098 w1101] -> w1092
                                tunnel: w1089 -> [_ w1100]
                                frame False {
                                }
                                frame True {
                                n800 = call <instrlib>:"TL4000 Set Laser Diode Current Setpoint.vi"("error in (no error)"=w1103, "Laser Diode Current Setpoint (0.0)"=w1100, "instrument handle"=w1104) -> ("error out"=w1101:errorcluster, "instrument handle out"=w1102:refnum<visa-resource-name>)  [unwired: 7 in]
                                }
                                }
                                }
                                frame #1 {
                                n801 = Wait (ms)(milliseconds to wait=u32 500) -> ()  [unwired: 1 out]
                                }
                                frame #2 {
                                n802 = call <instrlib>:"TLPM Measure Power.vi"("error in (no error)"=w1109, "instrument handle"=w1110) -> ("error out"=w1107:errorcluster, "Power"=w1106:dbl, "instrument handle out"=w1108:refnum<visa-resource-name>)  [unwired: 7 in]
                                n803 = local write "Excitation Power (uW)"(w1106) -> ()
                                }
                                }
                                n804 = Insert Into Array(array=w1079, new element=w1078) -> (w1077:dbl[])  [unwired: 1 in]
                                n805 = local write "Diode Driver Error out"(w1088) -> ()
                                n806 = local write "Photodiode handle out"(w1087) -> ()
                                n807 = local write "Photodiode error out"(w1085) -> ()
                                n808 = local write "Diode Driver COM"(w1086) -> ()
                                }
                                frame #1 {
                                # "open shutter if closed"
                                n809 = control-ref of="KCube Shutter Device Reference"() -> (w1115:refnum<vi>)
                                n810 = control-ref of="Shutter Ctrls"() -> (w1114:refnum<vi>)
                                n811 = property class="Ring (strict)"(reference=w1114) -> ("Value"=w1116:u16)  [unwired: 1 in, 2 out]
                                n812 = local read "KCube Shutter On?"() -> (w1119:bool)
                                n813 = Equal?(x=w1116, y=u16 0) -> (x = y?=w1118:bool)
                                n814 = property on="Experiment Graph Controls" class="TabCtl (strict)"("Value"=T25."Spectrum" ("Experiment Graph Controls")) -> ()  [unwired: 2 in, 2 out]
                                n815 = case shown="True" w1118 {
                                tunnel: w1115 -> [_ w1122]
                                tunnel: w1114 -> [_ w1121]
                                tunnel: w1119 -> [_ w1120]
                                frame False {
                                }
                                frame True {
                                n816 = call "Shutter.vi"("KCube Shutter Device Reference 2"=w1122, "Shutter Ctrls 2"=w1121, "Shutter on?"=w1120) -> ()
                                }
                                }
                                }
                                frame #2 {
                                # "set CCD ROI and acquire"
                                n817 = local read "LightField Automation error out"() -> (w1131:errorcluster)
                                n818 = local read "LightField Automation out"() -> (w1123:refnum<class "LightField Automation.lvclass">)
                                n819 = local read "CCD ROI"() -> (w1130:T20)
                                n820 = local read "Accumulations"() -> (w1127:dbl)
                                n821 = call "Adv_SetROI.vi"("error in (no error)"=w1131, "ROI"=w1130, "LightField Automation in"=w1123) -> ("error out"=w1128:errorcluster, "LightField Automation out"=w1129:refnum<class "LightField Automation.lvclass">)  [unwired: 7 in]
                                n822 = call "LFA_Capture.vi"("error in (no error)"=w1128, "Frames"=w1127, "LightField Automation in"=w1129) -> ("error out"=w1126:errorcluster, "Data"=w1125:T26, "LightField Automation out"=w1124:refnum<class "LightField Automation.lvclass">)  [unwired: 6 in]
                                n823 = local write "LightField Automation out"(w1124) -> ()
                                n824 = local write "LightField Automation error out"(w1126) -> ()
                                n825 = local write "Data"(w1125) -> ()
                                }
                                frame #3 {
                                # "close shutter"
                                n826 = local read "KCube Shutter On?"() -> (w1134:bool)
                                n827 = control-ref of="KCube Shutter Device Reference"() -> (w1133:refnum<vi>)
                                n828 = control-ref of="Shutter Ctrls"() -> (w1132:refnum<vi>)
                                n829 = call "Shutter.vi"("KCube Shutter Device Reference 2"=w1133, "Shutter Ctrls 2"=w1132, "Shutter on?"=w1134) -> ()
                                }
                                frame #4 {
                                # "Show data accordingly"
                                n830 = local read "Data"() -> (w1138:T26)
                                n831 = local read "Acq Mode"() -> (w1139:T3)
                                n832 = case shown="\"Spectrum\", Default" w1139 {
                                selector: w1139 -> [w1141 w1163]
                                tunnel: w1138 -> [w1142 w1164]
                                tunnel: [w1140 w1162] -> w1136
                                frame "Spectrum", Default {
                                n833 = stacked-sequence {
                                tunnel: w1142 -> [_ w1158 _]
                                tunnel: w1141 -> [_ w1156 _]
                                tunnel: [_ w1145 _] -> w1140
                                frame #0 {
                                n834 = property on="CCD 1D Spectrum Main" class="XYGraph (strict)"("Visible"=TRUE) -> ()  [unwired: 2 in, 2 out]
                                n835 = property on="CCD 2D Image Main" class="IntGraph (strict)"("Visible"=FALSE) -> ()  [unwired: 2 in, 2 out]
                                }
                                frame #1 {
                                n836 = local read "Wavelength calibration"() -> (w1155:dbl[])
                                n837 = local read "CCD ROI"() -> (w1151:T20)
                                n838 = Divide(x=1239.842, y=w1155) -> (x/y=w1153:dbl[])
                                n839 = call "PrepareData4Graph.vi"("Wavelength nm"=w1153, "DataLF"=w1158, "CCD ROI"=w1151, "AcqMode"=w1156, "Data type"=T30."Spectre") -> ("Spectrum"=w1157:cluster{"Array 2":dbl[], "Array":dbl[]}, "PLInt out"=w1145:dbl[])  [unwired: 2 in, 2 out]
                                n840 = local write "CCD 1D Spectrum Main"(w1157) -> ()
                                n841 = local read "Excitation Power (uW)"() -> (w1147:dbl)
                                n842 = local read "Acq Time (ms)"() -> (w1148:dbl)
                                n843 = local read "BackgroundSpec"() -> (w1146:dbl[])
                                n844 = local read "Display Mode"() -> (w1149:u16)
                                n845 = control-ref of="Cnts"() -> (w1150:refnum<vi>)
                                n846 = call "2Cnts.vi"("Array Background"=w1146, "Pow W"=w1147, "AcqTime ms"=w1148, "Cnts Ref"=w1150, "Display Mode"=w1149, "Array"=w1145) -> ()  [unwired: 1 out]
                                }
                                frame #2 {
                                n847 = property on="CCD 1D Spectrum Main" class="XYGraph (strict)"() -> ("Value"=w1161:cluster{dbl[], dbl[]})  [unwired: 2 in, 2 out]
                                n848 = Unbundle(w1161) -> (w1160:dbl[])  [unwired: 1 out]
                                n849 = call "myMax.vi"("Array"=w1160) -> ("myMax"=w1159:dbl)  [unwired: 1 in]
                                n850 = property on="CCD 1D Spectrum Main" class="XYGraph (strict)"("YScale.Maximum"=w1159) -> ()  [unwired: 2 in, 2 out]
                                }
                                }
                                }
                                frame "Image" {
                                n851 = stacked-sequence {
                                tunnel: w1164 -> [_ w1178]
                                tunnel: w1163 -> [_ w1176]
                                tunnel: [_ w1167] -> w1162
                                frame #0 {
                                n852 = property on="CCD 1D Spectrum Main" class="XYGraph (strict)"("Visible"=FALSE) -> ()  [unwired: 2 in, 2 out]
                                n853 = property on="CCD 2D Image Main" class="IntGraph (strict)"("Visible"=TRUE) -> ()  [unwired: 2 in, 2 out]
                                }
                                frame #1 {
                                n854 = local read "Wavelength calibration"() -> (w1177:dbl[])
                                n855 = local read "CCD ROI"() -> (w1173:T20)
                                n856 = call "PrepareData4Graph.vi"("Wavelength nm"=w1177, "DataLF"=w1178, "CCD ROI"=w1173, "AcqMode"=w1176, "Data type"=T30."Spectre") -> ("Intensity Graph"=w1175:dbl[][], "PLInt out"=w1167:dbl[])  [unwired: 2 in, 2 out]
                                n857 = local write "CCD 2D Image Main"(w1175) -> ()
                                n858 = local read "Excitation Power (uW)"() -> (w1169:dbl)
                                n859 = local read "Acq Time (ms)"() -> (w1170:dbl)
                                n860 = local read "BackgroundSpec"() -> (w1168:dbl[])
                                n861 = local read "Display Mode"() -> (w1171:u16)
                                n862 = control-ref of="Cnts"() -> (w1172:refnum<vi>)
                                n863 = call "2Cnts.vi"("Array Background"=w1168, "Pow W"=w1169, "AcqTime ms"=w1170, "Cnts Ref"=w1172, "Display Mode"=w1171, "Array"=w1167) -> ()  [unwired: 1 out]
                                }
                                }
                                }
                                }
                                n864 = Insert Into Array(array=w1137, new element=w1136) -> (w1135:i32[][])  [unwired: 2 in]
                                }
                                frame #5 {
                                n865 = local write "Scan Main Progess Bar"(w1179) -> ()
                                n866 = while {
                                stop <- w1180 continue-if-true
                                n867 = Wait (ms)(milliseconds to wait=u32 50) -> ()  [unwired: 1 out]
                                n868 = local read "MasterPause"() -> (w1180:bool)
                                }